vi "Controle_Manip_Main_GUI_WorkingBackup_211222.vi"() -> ()   [LabVIEW 2019] (continued)
                          frame #2 {
                            w3390 = T29."Enabled" ("Disabled")
                            n2748 = property on="Center Wavelength (nm)" class="DigNum (strict)"("DisabledEnum"=w3390) -> ()  [unwired: 2 in, 2 out]
                            n2749 = property on="Grating" class="CmbBox"("DisabledEnum"=w3390) -> ()  [unwired: 2 in, 2 out]
                            n2750 = property on="Exit mirror" class="Ring (strict)"("DisabledEnum"=w3390) -> ()  [unwired: 2 in, 2 out]
                          }
                        }
                      }
                      frame True {
                        n2751 = local write "LightField Automation error out"(w3391) -> ()
                        n2752 = local write "LightField Automation out"(w3392) -> ()
                      }
                    }
                  }
                }
              }
            }
          }
          event "Conv/Energy (eV)", "Conv/Wavelength (nm)", "Conv/Time (s)", "Conv/Wavenumber (m-1)": Value Change {
            n2753 = event-data() -> ("CtlRef"=w3395:refnum<vi>, "NewVal"=w3393:dbl)  [unwired: 1 in, 4 out]
            n2754 = property class="DigNum (strict)"(reference=w3395) -> ("Label.Text"=w3394:string)  [unwired: 1 in, 2 out]
            n2755 = case shown="\"Conv/Energy (eV)\"" w3394 {
              tunnel: w3393 -> [w3403 _ w3416 _]
              frame "Conv/Wavelength (nm)", Default {
                n2756 = Multiply(x=w3403, y=1e-09) -> (x*y=w3401:dbl)
                n2757 = Divide(x=1.0, y=w3401) -> (x/y=w3398:dbl)
                n2758 = Divide(x=w3401, y=299792458.0) -> (x/y=w3400:dbl)
                n2759 = Divide(x=w3398, y=100.0) -> (x/y=w3396:dbl)
                n2760 = Divide(x=1239.842, y=w3403) -> (x/y=w3405:dbl)
                n2761 = local write "Conv/Energy (eV)"(w3405) -> ()
                n2762 = local write "Conv/Wavenumber (m-1)"(w3396) -> ()
                n2763 = local write "Conv/Time (s)"(w3400) -> ()
              }
              frame "Conv/Time (s)" {
              }
              frame "Conv/Energy (eV)" {
                n2764 = Divide(x=1239.842, y=w3416) -> (x/y=w3415:dbl)
                n2765 = Multiply(x=w3415, y=1e-09) -> (x*y=w3412:dbl)
                n2766 = local write "Conv/Wavelength (nm)"(w3415) -> ()
                n2767 = Divide(x=1.0, y=w3412) -> (x/y=w3409:dbl)
                n2768 = Divide(x=w3409, y=100.0) -> (x/y=w3407:dbl)
                n2769 = Divide(x=w3412, y=299792458.0) -> (x/y=w3410:dbl)
                n2770 = local write "Conv/Wavenumber (m-1)"(w3407) -> ()
                n2771 = local write "Conv/Time (s)"(w3410) -> ()
              }
              frame "Conv/Wavenumber (m-1)" {
              }
            }
          }
          event "CCD ROI": Value Change {
            n2772 = event-data() -> ()  [unwired: 1 in, 6 out]
            n2773 = local read "LightField On?"() -> (w3418:bool)
            n2774 = case shown="True" w3418 {
              frame False {
              }
              frame True {
                n2775 = stacked-sequence {
                  frame #0 {
                    n2776 = property on="CCD ROI" class="Enum (strict)"("DisabledEnum"=T29."Disabled and Grayed Out" ("Disabled")) -> ()  [unwired: 2 in, 2 out]
                  }
                  frame #1 {
                    n2777 = local read "LightField Automation error out"() -> (w3422:errorcluster)
                    n2778 = local read "LightField Automation out"() -> (w3424:refnum<class "LightField Automation.lvclass">)
                    n2779 = local read "CCD ROI"() -> (w3423:T20)
                    n2780 = call "Adv_SetROI.vi"("error in (no error)"=w3422, "ROI"=w3423, "LightField Automation in"=w3424) -> ("error out"=w3421:errorcluster, "LightField Automation out"=w3420:refnum<class "LightField Automation.lvclass">)  [unwired: 7 in]
                    n2781 = local write "LightField Automation out"(w3420) -> ()
                    n2782 = local write "LightField Automation error out"(w3421) -> ()
                  }
                  frame #2 {
                    n2783 = property on="CCD ROI" class="Enum (strict)"("DisabledEnum"=T29."Enabled" ("Disabled")) -> ()  [unwired: 2 in, 2 out]
                  }
                }
              }
            }
          }
          event "Cryostat": Value Change {
            n2784 = event-data() -> ("NewVal"=w3426:enum16{"Montana", "Oxford"})  [unwired: 1 in, 5 out]
            n2785 = case shown="\"Montana\"" w3426 {
              frame "Oxford" {
                w3427 = FALSE
                n2786 = property on="FSM Up" class="Bool (strict)"("Visible"=w3427) -> ()  [unwired: 2 in, 2 out]
                n2787 = property on="FSM Left" class="Bool (strict)"("Visible"=w3427) -> ()  [unwired: 2 in, 2 out]
                n2788 = property on="FSM Axis Step" class="DigNum (strict)"("Visible"=w3427) -> ()  [unwired: 2 in, 2 out]
                n2789 = property on="FSM Down" class="Bool (strict)"("Visible"=w3427) -> ()  [unwired: 2 in, 2 out]
                n2790 = property on="FSM Right" class="Bool (strict)"("Visible"=w3427) -> ()  [unwired: 2 in, 2 out]
              }
              frame "Montana" {
                w3428 = TRUE
                n2791 = property on="FSM Up" class="Bool (strict)"("Visible"=w3428) -> ()  [unwired: 2 in, 2 out]
                n2792 = property on="FSM Left" class="Bool (strict)"("Visible"=w3428) -> ()  [unwired: 2 in, 2 out]
                n2793 = property on="FSM Axis Step" class="DigNum (strict)"("Visible"=w3428) -> ()  [unwired: 2 in, 2 out]
                n2794 = property on="FSM Down" class="Bool (strict)"("Visible"=w3428) -> ()  [unwired: 2 in, 2 out]
                n2795 = property on="FSM Right" class="Bool (strict)"("Visible"=w3428) -> ()  [unwired: 2 in, 2 out]
              }
            }
          }
          event "Excitation Power (uW)": Mouse Down; "Excitation Wavelength (nm)", "Excitation Source": Value Change {
            n2796 = event-data() -> ("CtlRef"=w3432:refnum<vi>)  [unwired: 1 in, 3 out]
            n2797 = property class="Num"(reference=w3432) -> ("Label.Text"=w3431:string)  [unwired: 1 in, 2 out]
            n2798 = case shown="\"Excitation Source\"" w3431 {
              tunnel: [w3433 w3434 w3445 w3470] -> w3429
              frame "False", Default {
                n2799 = local read "Excitation Wavelength (nm)"() -> (w3433:dbl)
              }
              frame "Excitation Power (uW)" {
                n2800 = local read "PM16-120 On?"() -> (w3435:bool)
                n2801 = case shown="True" w3435 {
                  tunnel: [w3436 w3437] -> w3434
                  frame False {
                    n2802 = local read "Excitation Wavelength (nm)"() -> (w3436:dbl)
                  }
                  frame True {
                    n2803 = local read "Excitation Wavelength (nm)"() -> (w3437:dbl)
                    n2804 = local read "Photodiode handle out"() -> (w3444:refnum<visa-resource-name>)
                    n2805 = local read "Photodiode error out"() -> (w3443:errorcluster)
                    n2806 = call <instrlib>:"TLPM Set Wavelength.vi"("error in (no error)"=w3443, "Wavelength (0.0)"=w3437, "instrument handle"=w3444) -> ("error out"=w3442:errorcluster, "instrument handle out"=w3441:refnum<visa-resource-name>)  [unwired: 7 in]
                    n2807 = call <instrlib>:"TLPM Measure Power.vi"("error in (no error)"=w3442, "instrument handle"=w3441) -> ("error out"=w3438:errorcluster, "Power"=w3440:dbl, "instrument handle out"=w3439:refnum<visa-resource-name>)  [unwired: 7 in]
                    n2808 = local write "Photodiode handle out"(w3439) -> ()
                    n2809 = local write "Photodiode error out"(w3438) -> ()
                    n2810 = local write "Excitation Power (uW)"(w3440) -> ()
                  }
                }
              }
              frame "Excitation Wavelength (nm)" {
                n2811 = stacked-sequence {
                  tunnel: [_ w3457] -> w3445
                  frame #0 {
                    n2812 = local read "Excitation Source"() -> (w3449:enum16{"P", "CW", "SK"})
                    n2813 = local read "LLTF On?"() -> (w3450:bool)
                    n2814 = Equal?(x=w3449, y=enum16{"P", "CW", "SK"}."SK") -> (x = y?=w3447:bool)
                    n2815 = And(x=w3450, y=w3447) -> (x .and. y?=w3446:bool)
                    n2816 = case shown="True" w3446 {
                      frame False {
                      }
                      frame True {
                        n2817 = local read "Excitation Wavelength (nm)"() -> (w3456:dbl)
                        n2818 = local read "LLTFDevice Interface"() -> (w3455:refnum<k7>)
                        n2819 = call "testmove.vi"("p_TargetWavelength"=w3456, "reference"=w3455) -> ("CurrentWavelength"=w3453:dbl, "CurrentAngle"=w3454:dbl, "Device reference out"=w3452:refnum<k7>, "Device moved"=w3451:bool)  [unwired: 4 in, 2 out]
                        n2820 = local write "LLTFDevice Interface"(w3452) -> ()
                        n2821 = local write "Device moved"(w3451) -> ()
                        n2822 = local write "CurrentAngle"(w3454) -> ()
                        n2823 = local write "CurrentWL"(w3453) -> ()
                      }
                    }
                  }
                  frame #1 {
                    n2824 = local read "PM16-120 On?"() -> (w3458:bool)
                    n2825 = case shown="True" w3458 {
                      tunnel: [w3459 w3460] -> w3457
                      frame False {
                        n2826 = local read "Excitation Wavelength (nm)"() -> (w3459:dbl)
                      }
                      frame True {
                        n2827 = local read "Excitation Wavelength (nm)"() -> (w3460:dbl)
                        n2828 = local read "Photodiode handle out"() -> (w3467:refnum<visa-resource-name>)
                        n2829 = local read "Photodiode error out"() -> (w3466:errorcluster)
                        n2830 = call <instrlib>:"TLPM Set Wavelength.vi"("error in (no error)"=w3466, "Wavelength (0.0)"=w3460, "instrument handle"=w3467) -> ("error out"=w3465:errorcluster, "instrument handle out"=w3464:refnum<visa-resource-name>)  [unwired: 7 in]
                        n2831 = call <instrlib>:"TLPM Measure Power.vi"("error in (no error)"=w3465, "instrument handle"=w3464) -> ("error out"=w3461:errorcluster, "Power"=w3463:dbl, "instrument handle out"=w3462:refnum<visa-resource-name>)  [unwired: 7 in]
                        n2832 = local write "Photodiode handle out"(w3462) -> ()
                        n2833 = local write "Photodiode error out"(w3461) -> ()
                        n2834 = local write "Excitation Power (uW)"(w3463) -> ()
                      }
                    }
                  }
                }
              }
              frame "Excitation Source" {
                n2835 = local read "Excitation Source"() -> (w3469:enum16{"P", "CW", "SK"})
                n2836 = local read "PM16-120 On?"() -> (w3471:bool)
                n2837 = case shown="Default" w3469 {
                  tunnel: [TRUE ("Laser on?") w3474] -> w3468
                  frame Default {
                  }
                  frame "CW" {
                    n2838 = local read "Laser on? Control"() -> (w3474:bool)
                    n2839 = local write "Excitation Wavelength (nm)"(448.5 ("Excitation Wavelength (nm)")) -> ()
                  }
                }
                n2840 = case shown="True" w3471 {
                  tunnel: [w3475 w3476] -> w3470
                  frame False {
                    n2841 = local read "Excitation Wavelength (nm)"() -> (w3475:dbl)
                  }
                  frame True {
                    n2842 = local read "Excitation Wavelength (nm)"() -> (w3476:dbl)
                    n2843 = local read "Photodiode handle out"() -> (w3483:refnum<visa-resource-name>)
                    n2844 = local read "Photodiode error out"() -> (w3482:errorcluster)
                    n2845 = call <instrlib>:"TLPM Set Wavelength.vi"("error in (no error)"=w3482, "Wavelength (0.0)"=w3476, "instrument handle"=w3483) -> ("error out"=w3481:errorcluster, "instrument handle out"=w3480:refnum<visa-resource-name>)  [unwired: 7 in]
                    n2846 = call <instrlib>:"TLPM Measure Power.vi"("error in (no error)"=w3481, "instrument handle"=w3480) -> ("error out"=w3477:errorcluster, "Power"=w3479:dbl, "instrument handle out"=w3478:refnum<visa-resource-name>)  [unwired: 7 in]
                    n2847 = local write "Photodiode handle out"(w3478) -> ()
                    n2848 = local write "Photodiode error out"(w3477) -> ()
                    n2849 = local write "Excitation Power (uW)"(w3479) -> ()
                  }
                }
                n2850 = local write "Laser on?"(w3468) -> ()
              }
            }
            n2851 = control-ref of="Laser on?"() -> (w3430:refnum<vi>)
            n2852 = call "ExcWL2LaserrColor.vi"("Wavelength (380 - 780)"=w3429, "Laser on?"=w3430) -> ()  [unwired: 1 in]
          }
          event "Exit mirror": Value Change {
            n2853 = event-data() -> ("NewVal"=w3484:u16)  [unwired: 1 in, 5 out]
            n2854 = local read "LightField On?"() -> (w3485:bool)
            n2855 = case shown="True" w3485 {
              tunnel: w3484 -> [_ w3492]
              frame False {
              }
              frame True {
                n2856 = stacked-sequence {
                  tunnel: w3492 -> [_ w3498 _]
                  tunnel: [_ w3497 _] -> w3487
                  tunnel: [_ w3496 _] -> w3486
                  frame #0 {
                    n2857 = control-ref of="Exit mirror"() -> (w3495:refnum<vi>)
                    n2858 = Build Array(w3495) -> (w3494:refnum<vi>[])
                    n2859 = call "Enable&Disable_Controls.vi"("Enum"=enum16{"Enabled", "Disabled", "Disabled&Grayed"}."Disabled&Grayed", "References"=w3494) -> ()  [unwired: 1 in]
                  }
                  frame #1 {
                    n2860 = case shown="4, Default" w3498 {
                      tunnel: [enum16{"Enabled", "Disabled", "Disabled&Grayed"}."Disabled&Grayed" ("Enum") enum16{"Enabled", "Disabled", "Disabled&Grayed"}."Enabled" ("Enum")] -> w3497
                      tunnel: [AcqMode."APD 1" ("Acq Mode") w3512] -> w3496
                      frame 5 {
                      }
                      frame 4, Default {
                        n2861 = property on="Acq Mode" class="Enum (strict)"() -> ("Value"=w3511:T3)  [unwired: 2 in, 2 out]
                        n2862 = Not Equal?(x=w3511, y=AcqMode."Image" ("Acq Mode")) -> (x != y?=w3509:bool)
                        n2863 = case shown="True" w3509 {
                          tunnel: [AcqMode."Image" ("Acq Mode") AcqMode."Spectrum" ("Acq Mode")] -> w3512
                          frame False {
                          }
                          frame True {
                          }
                        }
                      }
                    }
                    n2864 = local read "LightField Automation error out"() -> (w3506:errorcluster)
                    n2865 = local read "LightField Automation out"() -> (w3505:refnum<class "LightField Automation.lvclass">)
                    n2866 = call "spec_GetOpticalExitPort.vi"("error in (no error)"=w3506, "LightField Automation in"=w3505) -> ("error out"=w3503:errorcluster, "Exit Port Location"=w3502:T33, "LightField Automation out"=w3504:refnum<class "LightField Automation.lvclass">)  [unwired: 7 in]
                    n2867 = Equal?(x=w3502, y=w3498) -> (x = y?=w3501:bool)
                    n2868 = case shown="False" w3501 {
                      tunnel: w3504 -> [w3526 w3528]
                      tunnel: w3503 -> [w3525 w3527]
                      tunnel: w3498 -> [w3524 _]
                      tunnel: [w3517 w3528] -> w3500
                      tunnel: [w3516 w3527] -> w3499
                      frame False {
                        n2869 = call "spec_SetOpticalExitPort.vi"("error in (no error)"=w3525, "Exit Port Location"=w3524, "LightField Automation in"=w3526) -> ("error out"=w3519:errorcluster, "LightField Automation out"=w3518:refnum<class "LightField Automation.lvclass">)  [unwired: 7 in]
                        n2870 = call "spec_GetCenterWavelength.vi"("error in (no error)"=w3519, "LightField Automation in"=w3518) -> ("error out"=w3522:errorcluster, "Center Wavelength"=w3520:dbl, "LightField Automation out"=w3521:refnum<class "LightField Automation.lvclass">)  [unwired: 7 in]
                        n2871 = local write "Center Wavelength (nm)"(w3520) -> ()
                        n2872 = call "spec_getCalibration.vi"("error in (no error)"=w3522, "LightField Automation in"=w3521) -> ("error out"=w3516:errorcluster, "ColumnCalibration"=w3523:dbl[], "LightField Automation out"=w3517:refnum<class "LightField Automation.lvclass">)  [unwired: 7 in]
                        n2873 = local write "Wavelength calibration"(w3523) -> ()
                      }
                      frame True {
                      }
                    }
                    n2874 = local write "LightField Automation error out"(w3499) -> ()
                    n2875 = local write "LightField Automation out"(w3500) -> ()
                  }
                  frame #2 {
                    n2876 = property on="Exit mirror" class="Ring (strict)"() -> ("RingText.Text"=w3533:string)  [unwired: 2 in, 2 out]
                    n2877 = local read "Log file"() -> (w3537:string)
                    n2878 = control-ref of="Exit mirror"() -> (w3532:refnum<vi>)
                    n2879 = Concatenate Strings("Exit mirror set to " ("Add to log file"), w3533) -> (w3534:string)
                    n2880 = call "Write2LogFile.vi"("Add to log file"=w3534, "Log file before"=w3537, "Checkbox"=FALSE) -> ("Log file after"=w3536:string)
                    n2881 = Build Array(w3532) -> (w3531:refnum<vi>[])
                    n2882 = call "Enable&Disable_Controls.vi"("Enum"=enum16{"Enabled", "Disabled", "Disabled&Grayed"}."Enabled", "References"=w3531) -> ()  [unwired: 1 in]
                    n2883 = local write "Log file"(w3536) -> ()
                  }
                }
                n2884 = control-ref of="Accumulations"() -> (w3489:refnum<vi>)
                n2885 = control-ref of="CCD ROI"() -> (w3490:refnum<vi>)
                n2886 = control-ref of="Exposure Time (ms)"() -> (w3491:refnum<vi>)
                n2887 = Build Array(w3489, w3490, w3491) -> (w3488:refnum<vi>[])
                n2888 = call "Enable&Disable_Controls.vi"("Enum"=w3487, "References"=w3488) -> ()  [unwired: 1 in]
                n2889 = property on="Acq Mode" class="Enum (strict)"("Value"=w3486) -> ()  [unwired: 2 in, 2 out]
              }
            }
          }
          event "Exposure Time (ms)", "Acquire N: N": Value Change {
            n2890 = event-data() -> ("CtlRef"=w3541:refnum<vi>, "NewVal"=w3538:dbl)  [unwired: 1 in, 4 out]
            n2891 = property class="DigNum (strict)"(reference=w3541) -> ("Label.Text"=w3540:string)  [unwired: 1 in, 2 out]
            n2892 = local read "LightField On?"() -> (w3539:bool)
            n2893 = case shown="\"Exposure Time (ms)\"" w3540 {
              tunnel: w3538 -> [w3543 w3545]
              tunnel: w3539 -> [_ w3546]
              frame "Acquire N: N", Default {
                n2894 = local read "Acq Time (ms)"() -> (w3542:dbl)
                n2895 = call "unnecessary_multiplication.vi"("N"=w3543, "AcqTime ms"=w3542) -> ("AcqTime Total (s)"=w3544:dbl)
                n2896 = local write "Duration"(w3544) -> ()
              }
              frame "Exposure Time (ms)" {
                n2897 = case shown="True" w3546 {
                  tunnel: w3545 -> [_ w3558]
                  frame False {
                  }
                  frame True {
                    n2898 = local read "LightField Automation error out"() -> (w3565:errorcluster)
                    n2899 = local read "LightField Automation out"() -> (w3564:refnum<class "LightField Automation.lvclass">)
                    n2900 = Divide(x=w3558, y=1000.0) -> (x/y=w3559:dbl)
                    n2901 = call "Exp_CCD_GetExposureTime.vi"("error in (no error)"=w3565, "LightField Automation in"=w3564) -> ("error out"=w3560:errorcluster, "Exposure Time (s)"=w3563:dbl, "LightField Automation out"=w3561:refnum<class "LightField Automation.lvclass">)  [unwired: 7 in]
                    n2902 = Equal?(x=w3563, y=w3559) -> (x = y?=w3562:bool)
                    n2903 = case shown="False" w3562 {
                      tunnel: w3561 -> [w3568 w3578]
                      tunnel: w3560 -> [w3567 w3577]
                      tunnel: w3559 -> [w3569 _]
                      tunnel: w3558 -> [_ _]
                      frame False {
                        n2904 = stacked-sequence {
                          tunnel: w3569 -> [_ w3573 _]
                          tunnel: w3568 -> [_ w3572 _]
                          tunnel: w3567 -> [_ w3571 _]
                          frame #0 {
                            n2905 = property on="Exposure Time (ms)" class="DigNum (strict)"("DisabledEnum"=T29."Disabled and Grayed Out" ("Disabled")) -> ()  [unwired: 2 in, 2 out]
                          }
                          frame #1 {
                            n2906 = call "Exp_CCD_SetExposureTime.vi"("error in (no error)"=w3571, "Exposure Time (s)"=w3573, "LightField Automation in"=w3572) -> ("error out"=w3574:errorcluster, "LightField Automation out"=w3575:refnum<class "LightField Automation.lvclass">)  [unwired: 7 in]
                            n2907 = local write "LightField Automation out"(w3575) -> ()
                            n2908 = local write "LightField Automation error out"(w3574) -> ()
                          }
                          frame #2 {
                            n2909 = property on="Exposure Time (ms)" class="DigNum (strict)"("DisabledEnum"=T29."Enabled" ("Disabled")) -> ()  [unwired: 2 in, 2 out]
                          }
                        }
                      }
                      frame True {
                        n2910 = local write "LightField Automation out"(w3578) -> ()
                        n2911 = local write "LightField Automation error out"(w3577) -> ()
                      }
                    }
                  }
                }
                n2912 = disable-structure shown="Disabled" {
                  disable-tunnel: w3545 -> [w3552 _]
                  frame Disabled {
                    n2913 = local read "Scan Y Num. Pts"() -> (w3554:dbl)
                    n2914 = local read "Scan X Num. Pts"() -> (w3555:dbl)
                    n2915 = Divide(x=w3552, y=1000.0) -> (x/y=w3550:dbl)
                    n2916 = Multiply(x=w3554, y=w3555) -> (x*y=w3556:dbl)
                    n2917 = Add(x=w3550, y=0.17) -> (x+y=w3549:dbl)
                    n2918 = Multiply(x=w3549, y=w3556) -> (x*y=w3557:dbl)
                    n2919 = local write "Expected (s)"(w3557) -> ()
                  }
                  frame Enabled {
                  }
                }
                n2920 = local write "Acq Time (ms)"(w3545) -> ()
                n2921 = local read "Acquire N: N"() -> (w3547:dbl)
                n2922 = call "unnecessary_multiplication.vi"("N"=w3547, "AcqTime ms"=w3545) -> ("AcqTime Total (s)"=w3548:dbl)
                n2923 = local write "Duration"(w3548) -> ()
              }
            }
          }
          event "FSM Home": Mouse Down {
            n2924 = event-data() -> ()  [unwired: 1 in, 6 out]
            n2925 = local read "FSM 300 On?"() -> (w3579:bool)
            n2926 = case shown="True" w3579 {
              frame False {
              }
              frame True {
                w3581 = 0.0 ("Target Value (V)")
                w3580 = 0.0 ("Target Value (V)")
                n2927 = local read "FSM Y Task"() -> (w3582:refnum<k21>)
                n2928 = local read "FSM X Task"() -> (w3583:refnum<k21>)
                n2929 = call "FSMGoTo.vi"("Target Value (V)"=w3580, "FSM Task"=w3583) -> ()  [unwired: 1 out]
                n2930 = call "FSMGoTo.vi"("Target Value (V)"=w3581, "FSM Task"=w3582) -> ()  [unwired: 1 out]
                n2931 = local write "Scan X Readout (V)"(w3580) -> ()
                n2932 = local write "Scan Y Readout (V)"(w3581) -> ()
                n2933 = property on="XY Intensity Map" class="IntGraph (strict)"("Cursor.Cursor X"=w3580) -> ()  [unwired: 2 in, 2 out]
                n2934 = property on="XY Intensity Map" class="IntGraph (strict)"("Cursor.Cursor Y"=w3581) -> ()  [unwired: 2 in, 2 out]
              }
            }
          }
          event "FSM Up", "FSM Down", "FSM Left", "FSM Right": Mouse Down {
            n2935 = event-data() -> ("CtlRef"=w3585:refnum<vi>)  [unwired: 1 in, 7 out]
            n2936 = local read "FSM 300 On?"() -> (w3584:bool)
            n2937 = case shown="True" w3584 {
              tunnel: w3585 -> [_ w3590]
              frame False {
              }
              frame True {
                n2938 = property class="Bool (strict)"(reference=w3590) -> ("Label.Text"=w3588:string)  [unwired: 1 in, 2 out]
                n2939 = local read "FSM Axis Step"() -> (w3589:dbl)
                n2940 = case shown="\"FSM Down\"" w3588 {
                  tunnel: [w3594 w3598 w3602 w3606] -> w3587
                  tunnel: w3589 -> [w3592 w3596 w3600 w3604]
                  tunnel: [w3591 w3595 w3599 w3603] -> w3586
                  frame "FSM Up", Default {
                    n2941 = local read "Scan Y Readout (V)"() -> (w3593:dbl)
                    n2942 = Add(x=w3593, y=w3592) -> (x+y=w3591:dbl)
                    n2943 = local write "Scan Y Readout (V)"(w3591) -> ()
                    n2944 = property on="XY Intensity Map" class="IntGraph (strict)"("Cursor.Cursor Y"=w3591) -> ()  [unwired: 2 in, 2 out]
                    n2945 = local read "FSM Y Task"() -> (w3594:refnum<k21>)
                  }
                  frame "FSM Down" {
                    n2946 = local read "Scan Y Readout (V)"() -> (w3597:dbl)
                    n2947 = Subtract(x=w3597, y=w3596) -> (x-y=w3595:dbl)
                    n2948 = local write "Scan Y Readout (V)"(w3595) -> ()
                    n2949 = local read "FSM Y Task"() -> (w3598:refnum<k21>)
                    n2950 = property on="XY Intensity Map" class="IntGraph (strict)"("Cursor.Cursor Y"=w3595) -> ()  [unwired: 2 in, 2 out]
                  }
                  frame "FSM Left" {
                    n2951 = local read "Scan X Readout (V)"() -> (w3601:dbl)
                    n2952 = Subtract(x=w3601, y=w3600) -> (x-y=w3599:dbl)
                    n2953 = local write "Scan X Readout (V)"(w3599) -> ()
                    n2954 = property on="XY Intensity Map" class="IntGraph (strict)"("Cursor.Cursor X"=w3599) -> ()  [unwired: 2 in, 2 out]
                    n2955 = local read "FSM X Task"() -> (w3602:refnum<k21>)
                  }
                  frame "FSM Right" {
                    n2956 = local read "Scan X Readout (V)"() -> (w3605:dbl)
                    n2957 = Add(x=w3605, y=w3604) -> (x+y=w3603:dbl)
                    n2958 = local write "Scan X Readout (V)"(w3603) -> ()
                    n2959 = property on="XY Intensity Map" class="IntGraph (strict)"("Cursor.Cursor X"=w3603) -> ()  [unwired: 2 in, 2 out]
                    n2960 = local read "FSM X Task"() -> (w3606:refnum<k21>)
                  }
                }
                n2961 = call "FSMGoTo.vi"("Target Value (V)"=w3586, "FSM Task"=w3587) -> ()  [unwired: 1 out]
              }
            }
          }
          event "FSM X Axis Pos", "FSM Y Axis Pos": Value Change {
            # "Move steering mirror"
            n2962 = event-data() -> ("CtlRef"=w3609:refnum<vi>, "NewVal"=w3608:dbl)  [unwired: 1 in, 4 out]
            n2963 = local read "FSM 300 On?"() -> (w3607:bool)
            n2964 = case shown="True" w3607 {
              tunnel: w3609 -> [_ w3613]
              tunnel: w3608 -> [_ w3610]
              frame False {
              }
              frame True {
                n2965 = property class="DigNum (strict)"(reference=w3613) -> ("Label.Text"=w3612:string)  [unwired: 1 in, 2 out]
                n2966 = case shown="\"FSM Y Axis Pos\"" w3612 {
                  tunnel: [w3615 w3617] -> w3611
                  tunnel: w3610 -> [w3614 w3616]
                  frame "FSM Y Axis Pos" {
                    n2967 = local write "Scan Y Readout (V)"(w3614) -> ()
                    n2968 = property on="XY Intensity Map" class="IntGraph (strict)"("Cursor.Cursor Y"=w3614) -> ()  [unwired: 2 in, 2 out]
                    n2969 = local read "FSM Y Task"() -> (w3615:refnum<k21>)
                  }
                  frame "FSM X Axis Pos", Default {
                    n2970 = local write "Scan X Readout (V)"(w3616) -> ()
                    n2971 = property on="XY Intensity Map" class="IntGraph (strict)"("Cursor.Cursor X"=w3616) -> ()  [unwired: 2 in, 2 out]
                    n2972 = local read "FSM X Task"() -> (w3617:refnum<k21>)
                  }
                }
                n2973 = call "FSMGoTo.vi"("Target Value (V)"=w3610, "FSM Task"=w3611) -> ()  [unwired: 1 out]
              }
            }
          }
          event "Add location": Mouse Down {
            (unwired) FALSE
            w3620 = "\r"
            n2974 = event-data() -> ()  [unwired: 1 in, 8 out]
            n2975 = local read "Map Marker X Pos"() -> (w3624:i8)
            n2976 = local read "Map Marker Y Pos"() -> (w3625:i8)
            n2977 = Format Into String(w3624) -> (resulting string=w3623:string)  [unwired: 3 in, 1 out]
            n2978 = Format Into String(w3625) -> (resulting string=w3621:string)  [unwired: 3 in, 1 out]
            n2979 = Concatenate Strings(w3620, "### Location ", w3623, "x" ("string"), w3621, w3620) -> (w3619:string)
            n2980 = call "Write2Markdown.vi"("String"=w3619) -> ()
            "ExportMapPosition?" <- FALSE ("ExportMapPosition?")
          }
          event "Full scale": Value Change {
            n2981 = event-data() -> ()  [unwired: 1 in, 6 out]
            n2982 = stacked-sequence {
              frame #0 {
                w3635 = 1239.842
                n2983 = property on="CCD 1D Spectrum Main" class="XYGraph (strict)"() -> ("Value"=w3630:cluster{dbl[], dbl[]})  [unwired: 2 in, 2 out]
                n2984 = Unbundle(w3630) -> (w3629:dbl[])  [unwired: 1 out]
                n2985 = property on="CCD 1D Spectrum Main" class="XYGraph (strict)"("XScale.ScaleFit"=u8 1 ("X Scale.Scale Fit"), "YScale.Minimum"=0.0 ("Y Scale.Range:Minimum")) -> ("XScale.Minimum"=w3627:dbl, "XScale.Maximum"=w3632:dbl)  [unwired: 2 in, 2 out]
                n2986 = call "myMax.vi"("Array"=w3629) -> ("myMax"=w3628:dbl)  [unwired: 1 in]
                n2987 = Divide(x=w3635, y=w3627) -> (x/y=w3633:dbl)
                n2988 = Divide(x=w3635, y=w3632) -> (x/y=w3634:dbl)
                n2989 = property on="CCD 1D Spectrum Main" class="XYGraph (strict)"("YScale.Maximum"=w3628) -> ()  [unwired: 2 in, 2 out]
                n2990 = property on="CCD 1D Spectrum Main Energy Scale" class="XYGraph (strict)"("XScale.Maximum"=w3633, "XScale.Minimum"=w3634) -> ()  [unwired: 2 in, 2 out]
              }
              frame #1 {
                n2991 = property on="Full scale" class="Bool (strict)"("Value"=FALSE ("Full scale")) -> ()  [unwired: 2 in, 2 out]
              }
            }
          }
          event "Grating": Value Change {
            n2992 = event-data() -> ("NewVal"=w3639:string)  [unwired: 1 in, 5 out]
            n2993 = local read "LightField On?"() -> (w3638:bool)
            n2994 = case shown="True" w3638 {
              tunnel: w3639 -> [_ w3646]
              frame False {
              }
              frame True {
                n2995 = local read "LightField Automation error out"() -> (w3645:errorcluster)
                n2996 = local read "LightField Automation out"() -> (w3643:refnum<class "LightField Automation.lvclass">)
                n2997 = call "spec_GetGratings.vi"("error in (no error)"=w3645, "LightField Automation in"=w3643) -> ("error out"=w3644:errorcluster, "Current Grating"=w3641:string, "LightField Automation out"=w3642:refnum<class "LightField Automation.lvclass">)  [unwired: 6 in, 1 out]
                n2998 = Equal?(x=w3646, y=w3641) -> (x = y?=w3640:bool)
                n2999 = case shown="False" w3640 {
                  tunnel: w3646 -> [w3652 _]
                  tunnel: w3644 -> [w3651 w3678]
                  tunnel: w3642 -> [w3650 w3679]
                  frame False {
                    n3000 = stacked-sequence {
                      seq-local: [_ w3662 _ _ _] -> [_ _ w3667 _ _]
                      seq-local: [_ w3661 _ _ _] -> [_ _ w3666 _ _]
                      seq-local: [_ w3660 _ _ _] -> [_ _ w3663 _ _]
                      seq-local: [_ _ w3665 _ _] -> [_ _ _ w3675 _]
                      seq-local: [_ _ w3664 _ _] -> [_ _ _ w3674 _]
                      seq-local: [_ _ w3663 _ _] -> [_ _ _ w3672 _]
                      tunnel: w3650 -> [_ w3662 _ _ _]
                      tunnel: w3651 -> [_ w3661 _ _ _]
                      tunnel: w3652 -> [_ w3660 _ _ _]
                      tunnel: [_ _ _ w3675 _] -> w3657
                      tunnel: [_ _ _ w3674 _] -> w3656
                      frame #0 {
                        n3001 = property on="Grating" class="CmbBox"("DisabledEnum"=T29."Disabled and Grayed Out" ("Disabled")) -> ()  [unwired: 2 in, 2 out]
                      }
                      frame #1 {
                      }
                      frame #2 {
                        n3002 = call "spec_SetGrating.vi"("error in (no error)"=w3666, "GratingSelected"=w3663, "LightField Automation in"=w3667) -> ("error out"=w3664:errorcluster, "LightField Automation out"=w3665:refnum<class "LightField Automation.lvclass">)  [unwired: 7 in]
                      }
                      frame #3 {
                        n3003 = local read "Log file"() -> (w3671:string)
                        n3004 = Concatenate Strings("Grating changed to " ("string"), w3672) -> (w3670:string)
                        n3005 = call "Write2LogFile.vi"("Add to log file"=w3670, "Log file before"=w3671, "Checkbox"=FALSE) -> ("Log file after"=w3669:string)
                        n3006 = local write "Log file"(w3669) -> ()
                      }
                      frame #4 {
                        n3007 = property on="Background substract" class="Enum (strict)"("Val(Sgnl)"=enum16{"None", "Shutter"}."Shutter" ("Value (Signaling)")) -> ()  [unwired: 2 in, 2 out]
                        n3008 = property on="Grating" class="CmbBox"("DisabledEnum"=T29."Enabled" ("Disabled")) -> ()  [unwired: 2 in, 2 out]
                      }
                    }
                    n3009 = call "spec_GetCenterWavelength.vi"("error in (no error)"=w3656, "LightField Automation in"=w3657) -> ("error out"=w3655:errorcluster, "Center Wavelength"=w3653:dbl, "LightField Automation out"=w3654:refnum<class "LightField Automation.lvclass">)  [unwired: 7 in]
                    n3010 = local write "Center Wavelength (nm)"(w3653) -> ()
                    n3011 = local write "Background taken?"(FALSE ("Background taken?")) -> ()
                    n3012 = call "spec_getCalibration.vi"("error in (no error)"=w3655, "LightField Automation in"=w3654) -> ("error out"=w3649:errorcluster, "ColumnCalibration"=w3658:dbl[], "LightField Automation out"=w3648:refnum<class "LightField Automation.lvclass">)  [unwired: 7 in]
                    n3013 = local write "LightField Automation out"(w3648) -> ()
                    n3014 = local write "LightField Automation error out"(w3649) -> ()
                    n3015 = local write "Wavelength calibration"(w3658) -> ()
                  }
                  frame True {
                    n3016 = local write "LightField Automation out"(w3679) -> ()
                    n3017 = local write "LightField Automation error out"(w3678) -> ()
                  }
                }
              }
            }
          }
          event "Mono2 On": Value Change {
            n3018 = event-data() -> ("NewVal"=w3681:bool)  [unwired: 1 in, 5 out]
            n3019 = local read "ESP 300 On?"() -> (w3680:bool)
            n3020 = case shown="True" w3680 {
              tunnel: w3681 -> [_ w3682]
              frame False {
              }
              frame True {
                n3021 = case shown="True" w3682 {
                  frame False {
                    n3022 = stacked-sequence {
                      frame #0 {
                        n3023 = local read "ESP300 COM Port"() -> (w3686:refnum<visa-resource-name>)
                        n3024 = local read "ESP300 Error"() -> (w3687:errorcluster)
                        n3025 = call "Motor Off.vi"("error in (no error)"=w3687, "Axis"=1, "VISA resource name in"=w3686) -> ("error out"=w3684:errorcluster, "VISA resource name out"=w3683:refnum<visa-resource-name>)  [unwired: 7 in]
                        n3026 = local write "ESP300 Error"(w3684) -> ()
                        n3027 = local write "ESP300 COM Port"(w3683) -> ()
                      }
                      frame #1 {
                        n3028 = local read "Log file"() -> (w3690:string)
                        n3029 = call "Write2LogFile.vi"("Add to log file"="Mono2 motor turned off", "Log file before"=w3690, "Checkbox"=FALSE) -> ("Log file after"=w3691:string)
                        n3030 = local write "Log file"(w3691) -> ()
                      }
                    }
                  }
                  frame True {
                    n3031 = stacked-sequence {
                      frame #0 {
                        n3032 = local read "ESP300 COM Port"() -> (w3695:refnum<visa-resource-name>)
                        n3033 = local read "ESP300 Error"() -> (w3696:errorcluster)
                        n3034 = call "Motor On.vi"("error in (no error)"=w3696, "Axis"=1, "VISA resource name in"=w3695) -> ("error out"=w3693:errorcluster, "VISA resource name out"=w3692:refnum<visa-resource-name>)  [unwired: 7 in]
                        n3035 = local write "ESP300 Error"(w3693) -> ()
                        n3036 = local write "ESP300 COM Port"(w3692) -> ()
                      }
                      frame #1 {
                        n3037 = local read "Log file"() -> (w3699:string)
                        n3038 = call "Write2LogFile.vi"("Add to log file"="Mono2 motor turned on", "Log file before"=w3699, "Checkbox"=FALSE) -> ("Log file after"=w3700:string)
                        n3039 = local write "Log file"(w3700) -> ()
                      }
                    }
                  }
                }
              }
            }
          }
          event "Motor LinT On?", "Motor RotStage Exc On?", "Motor RotStage Det On?", "LinTFine Motor On?": Mouse Down {
            n3040 = event-data() -> ("CtlRef"=w3703:refnum<vi>)  [unwired: 1 in, 7 out]
            n3041 = property class="Bool (strict)"(reference=w3703) -> ("Label.Text"=w3702:string, "Value"=w3701:bool)  [unwired: 1 in, 2 out]
            n3042 = case shown="\"LinTFine Motor On?\"" w3702 {
              tunnel: w3701 -> [w3705 _ w3713 w3721 w3729]
              frame "Motor RotStage Exc On?" {
                n3043 = local read "ESP 301 On?"() -> (w3704:bool)
                n3044 = case shown="True" w3704 {
                  tunnel: w3705 -> [_ w3706]
                  frame False {
                  }
                  frame True {
                    n3045 = local read "ESP 301 COM Port"() -> (w3711:refnum<visa-resource-name>)
                    n3046 = local read "ESP 301 Error"() -> (w3710:errorcluster)
                    n3047 = call "Enable Disable Motor.vi"("error in (no error)"=w3710, "Action (F - OFF)"=w3706, "Axis (1)"=2, "VISA resource name"=w3711) -> ("error out"=w3708:errorcluster, "VISA resource name out"=w3709:refnum<visa-resource-name>)  [unwired: 2 in]
                    n3048 = local write "ESP 301 COM Port"(w3709) -> ()
                    n3049 = local write "ESP 301 Error"(w3708) -> ()
                  }
                }
              }
              frame Default {
                # "default do nothing"
              }
              frame "LinTFine Motor On?" {
                n3050 = local read "PZC200 On?"() -> (w3712:bool)
                n3051 = case shown="True" w3712 {
                  tunnel: w3713 -> [_ w3716]
                  frame False {
                  }
                  frame True {
                    n3052 = case shown="False" w3716 {
                      tunnel: ["1MF" "1MO" ("Command")] -> w3715
                      frame False {
                      }
                      frame True {
                      }
                    }
                    n3053 = local read "PZC200 Instrument Channel"() -> (w3717:string)
                    n3054 = call "SendCommand.vi"("Command"=w3715, "Instrument Channel"=w3717) -> ("Instrument Channel out"=w3714:string)  [unwired: 8 in, 1 out]
                    n3055 = local write "PZC200 Instrument Channel"(w3714) -> ()
                  }
                }
              }
              frame "Motor LinT On?" {
                n3056 = local read "ESP 301 On?"() -> (w3720:bool)
                n3057 = case shown="True" w3720 {
                  tunnel: w3721 -> [_ w3724]
                  frame False {
                  }
                  frame True {
                    n3058 = local read "ESP 301 COM Port"() -> (w3727:refnum<visa-resource-name>)
                    n3059 = local read "ESP 301 Error"() -> (w3726:errorcluster)
                    n3060 = call "Enable Disable Motor.vi"("error in (no error)"=w3726, "Action (F - OFF)"=w3724, "Axis (1)"=1, "VISA resource name"=w3727) -> ("error out"=w3722:errorcluster, "VISA resource name out"=w3723:refnum<visa-resource-name>)  [unwired: 2 in]
                    n3061 = local write "ESP 301 COM Port"(w3723) -> ()
                    n3062 = local write "ESP 301 Error"(w3722) -> ()
                  }
                }
              }
              frame "Motor RotStage Det On?" {
                n3063 = local read "ESP 301 On?"() -> (w3728:bool)
                n3064 = case shown="True" w3728 {
                  tunnel: w3729 -> [_ w3730]
                  frame False {
                  }
                  frame True {
                    n3065 = local read "ESP 301 COM Port"() -> (w3735:refnum<visa-resource-name>)
                    n3066 = local read "ESP 301 Error"() -> (w3734:errorcluster)
                    n3067 = call "Enable Disable Motor.vi"("error in (no error)"=w3734, "Action (F - OFF)"=w3730, "Axis (1)"=3, "VISA resource name"=w3735) -> ("error out"=w3732:errorcluster, "VISA resource name out"=w3733:refnum<visa-resource-name>)  [unwired: 2 in]
                    n3068 = local write "ESP 301 COM Port"(w3733) -> ()
                    n3069 = local write "ESP 301 Error"(w3732) -> ()
                  }
                }
              }
            }
          }
          event "PZC Position Readout (usteps)", "RotStage Exc Angle Readout (°)", "RotStage Det Angle Readout (°)", "Newport Linear Translation Stage Position Readout (mm)": Mouse Down {
            n3070 = event-data() -> ("CtlRef"=w3738:refnum<vi>)  [unwired: 1 in, 7 out]
            n3071 = property class="DigNum (strict)"(reference=w3738) -> ("Label.Text"=w3737:string)  [unwired: 1 in, 2 out]
            n3072 = case shown="\"RotStage Det Angle Readout (°)\"" w3737 {
              tunnel: [0.0 ("Position (units)") w3740 w3751 w3762 w3769] -> w3736
              frame "False", Default {
              }
              frame "RotStage Exc Angle Readout (°)" {
                n3073 = local read "ESP 301 On?"() -> (w3741:bool)
                n3074 = case shown="True" w3741 {
                  tunnel: [0.0 ("Position (units)") w3748] -> w3740
                  frame False {
                  }
                  frame True {
                    w3743 = 3 ("Axis (1)")
                    n3075 = local read "ESP 301 COM Port"() -> (w3746:refnum<visa-resource-name>)
                    n3076 = local read "ESP 301 Error"() -> (w3747:errorcluster)
                    n3077 = call "Read absolute position.vi"("error in (no error)"=w3747, "Axis (1)"=w3743, "VISA resource name"=w3746) -> ("error out"=w3744:errorcluster, "VISA resource name out"=w3745:refnum<visa-resource-name>)  [unwired: 2 in, 1 out]
                    n3078 = call "Read absolute position.vi"("error in (no error)"=w3744, "Axis (1)"=w3743, "VISA resource name"=w3745) -> ("error out"=w3749:errorcluster, "Position (units)"=w3748:dbl, "VISA resource name out"=w3750:refnum<visa-resource-name>)  [unwired: 2 in]
                    n3079 = local write "ESP 301 COM Port"(w3750) -> ()
                    n3080 = local write "RotStage Exc Angle Readout (°)"(w3748) -> ()
                    n3081 = local write "ESP 301 Error"(w3749) -> ()
                  }
                }
              }
              frame "RotStage Det Angle Readout (°)" {
                n3082 = local read "ESP 301 On?"() -> (w3752:bool)
                n3083 = case shown="True" w3752 {
                  tunnel: [0.0 ("Position (units)") w3759] -> w3751
                  frame False {
                  }
                  frame True {
                    w3754 = 2 ("Axis (1)")
                    n3084 = local read "ESP 301 COM Port"() -> (w3755:refnum<visa-resource-name>)
                    n3085 = local read "ESP 301 Error"() -> (w3758:errorcluster)
                    n3086 = call "Read absolute position.vi"("error in (no error)"=w3758, "Axis (1)"=w3754, "VISA resource name"=w3755) -> ("error out"=w3757:errorcluster, "VISA resource name out"=w3756:refnum<visa-resource-name>)  [unwired: 2 in, 1 out]
                    n3087 = call "Read absolute position.vi"("error in (no error)"=w3757, "Axis (1)"=w3754, "VISA resource name"=w3756) -> ("error out"=w3761:errorcluster, "Position (units)"=w3759:dbl, "VISA resource name out"=w3760:refnum<visa-resource-name>)  [unwired: 2 in]
                    n3088 = local write "ESP 301 COM Port"(w3760) -> ()
                    n3089 = local write "RotStage Det Angle Readout (°)"(w3759) -> ()
                    n3090 = local write "ESP 301 Error"(w3761) -> ()
                  }
                }
              }
              frame "Newport Linear Translation Stage Position Readout (mm)" {
                n3091 = local read "ESP 301 On?"() -> (w3763:bool)
                n3092 = case shown="True" w3763 {
                  tunnel: [0.0 ("Position (units)") w3768] -> w3762
                  frame False {
                  }
                  frame True {
                    n3093 = local read "ESP 301 COM Port"() -> (w3766:refnum<visa-resource-name>)
                    n3094 = local read "ESP 301 Error"() -> (w3765:errorcluster)
                    n3095 = call "Read Actual Position.vi"("error in (no error)"=w3765, "Axis (1)"=1, "VISA resource name"=w3766) -> ("Position (units)"=w3768:dbl)  [unwired: 2 in, 2 out]
                    n3096 = local write "Newport Linear Translation Stage Position Readout (mm)"(w3768) -> ()
                  }
                }
              }
              frame "PZC Position Readout (usteps) " {
                n3097 = local read "PZC200 On?"() -> (w3770:bool)
                n3098 = case shown="True" w3770 {
                  tunnel: [0 ("Position") w3772] -> w3769
                  frame False {
                  }
                  frame True {
                    n3099 = local read "PZC200 Instrument Channel"() -> (w3775:string)
                    n3100 = call "PZCGetPos.vi"("Instrument Channel"=w3775) -> ("Instrument Channel Out"=w3773:string, "Position"=w3772:i32, "error out"=w3774:errorcluster)  [unwired: 1 in]
                    n3101 = local write "PZC Error"(w3774) -> ()
                    n3102 = local write "PZC Position Readout (usteps)"(w3772) -> ()
                    n3103 = local write "PZC200 Instrument Channel"(w3773) -> ()
                  }
                }
              }
            }
            "Position (units)" <- w3736
          }
          event "Reset origins": Value Change {
            n3104 = event-data() -> ("NewVal"=w3776:bool)  [unwired: 1 in, 5 out]
            n3105 = case shown="True" w3776 {
              frame False {
              }
              frame True {
                n3106 = disable-structure shown="Disabled" {
                  frame Disabled {
                    n3107 = local read "PZC Position Readout (usteps)"() -> ()  [unwired: 1 out]
                    n3108 = local read "Newport Linear Translation Stage Position Readout (mm)"() -> ()  [unwired: 1 out]
                  }
                  frame Enabled {
                  }
                }
              }
            }
          }
          event "RotStage Exc Angle (°)", "RotStage Det Angle (°)", "Newport Linear Translation Stage Position (mm)", "Newport PZA12 Stage Position (usteps)": Value Change {
            n3109 = event-data() -> ("CtlRef"=w3779:refnum<vi>, "NewVal"=w3778:dbl)  [unwired: 1 in, 4 out]
            n3110 = property class="DigNum (strict)"(reference=w3779) -> ("Label.Text"=w3777:string)  [unwired: 1 in, 2 out]
            n3111 = case shown="\"RotStage Exc Angle (°)\"" w3777 {
              tunnel: w3777 -> [_ _ w3798 _ w3838 w3867]
              tunnel: w3778 -> [_ w3781 w3797 w3833 w3837 w3866]
              frame "False", Default {
              }
              frame "Newport PZA12 Stage Position (usteps)" {
                n3112 = local read "PZC200 On?"() -> (w3780:bool)
                n3113 = case shown="True" w3780 {
                  tunnel: w3781 -> [_ w3783]
                  frame False {
                  }
                  frame True {
                    n3114 = local read "PZC200 Instrument Channel"() -> (w3787:string)
                    n3115 = call "PZCGetPos.vi"("Instrument Channel"=w3787) -> ("Instrument Channel Out"=w3784:string, "Position"=w3786:i32)  [unwired: 1 in, 1 out]
                    n3116 = Not Equal?(x=w3783, y=w3786) -> (x != y?=w3785:bool)
                    n3117 = case shown="True" w3785 {
                      tunnel: w3784 -> [w3788 w3791]
                      tunnel: w3783 -> [_ w3790]
                      tunnel: [w3788 w3789] -> w3782
                      frame False {
                      }
                      frame True {
                        n3118 = stacked-sequence {
                          tunnel: w3791 -> [w3795]
                          tunnel: w3790 -> [w3794]
                          tunnel: [w3792] -> w3789
                          frame #0 {
                            n3119 = call "PZC_MoveAbs.vi"("Target"=w3794, "Instrument"=w3795) -> ("Final Position"=w3793:i32, "Instrument out"=w3792:string)  [unwired: 1 in, 1 out]
                            n3120 = local write "PZC Position Readout (usteps)"(w3793) -> ()
                          }
                        }
                      }
                    }
                    n3121 = local write "PZC200 Instrument Channel"(w3782) -> ()
                  }
                }
              }
              frame "Newport Linear Translation Stage Position (mm)" {
                n3122 = local read "ESP 301 On?"() -> (w3796:bool)
                n3123 = case shown="True" w3796 {
                  tunnel: w3798 -> [_ w3813]
                  tunnel: w3797 -> [_ w3802]
                  frame False {
                  }
                  frame True {
                    n3124 = case shown="\"Newport Linear Translation Stage Position (mm)\"" w3813 {
                      tunnel: [2 1 3] -> w3814
                      tunnel: [w3817 w3820 w3823] -> w3811
                      tunnel: w3802 -> [w3816 w3819 w3822]
                      frame "RotStage Det Angle (°)" {
                        n3125 = local write "RotStage Det Angle (°)"(w3816) -> ()
                        n3126 = control-ref of="RotStage Det Angle Readout (°)"() -> (w3817:refnum<vi>)
                      }
                      frame "Newport Linear Translation Stage Position (mm)" {
                        n3127 = control-ref of="Newport Linear Translation Stage Position Readout (mm)"() -> (w3820:refnum<vi>)
                        n3128 = local write "Newport Linear Translation Stage Position (mm)"(w3819) -> ()
                      }
                      frame "RotStage Exc Angle (°)", Default {
                        n3129 = local write "RotStage Exc Angle (°)"(w3822) -> ()
                        n3130 = control-ref of="RotStage Exc Angle Readout (°)"() -> (w3823:refnum<vi>)
                      }
                    }
                    n3131 = local read "Excitation Wavelength (nm)"() -> (w3807:dbl)
                    n3132 = local read "Photodiode Status"() -> (w3799:bool)
                    n3133 = local read "Photodiode handle out"() -> (w3809:refnum<visa-resource-name>)
                    n3134 = local read "Photodiode error out"() -> (w3808:errorcluster)
                    n3135 = local read "ESP 301 Error"() -> (w3815:errorcluster)
                    n3136 = control-ref of="Excitation Power (uW)"() -> (w3810:refnum<vi>)
                    n3137 = call <instrlib>:"TLPM Set Wavelength.vi"("error in (no error)"=w3808, "Wavelength (0.0)"=w3807, "instrument handle"=w3809) -> ("error out"=w3805:errorcluster, "instrument handle out"=w3806:refnum<visa-resource-name>)  [unwired: 7 in]
                    n3138 = local read "ESP 301 COM Port"() -> (w3801:refnum<visa-resource-name>)
                    n3139 = call "Go2Angle.vi"("VISA resource name"=w3801, "Photodiode"=w3806, "RotStage Det Angle Readout (°) 4"=w3811, "Excitation Power (uW) 2"=w3810, "Photodiode on?"=w3799, "Axis ESP301 / RotStage"=w3814, "ESP301 Error"=w3815, "Photodiode error"=w3805, "Position (units)"=w3802) -> ("Photodiode out"=w3803:refnum<visa-resource-name>, "VISA resource name out"=w3800:refnum<visa-resource-name>, "Photodiode"=w3804:errorcluster, "ESP301 Error out"=w3812:errorcluster)  [unwired: 3 in]
                    n3140 = local write "ESP 301 Error"(w3812) -> ()
                    n3141 = local write "Photodiode handle out"(w3803) -> ()
                    n3142 = local write "Photodiode error out"(w3804) -> ()
                    n3143 = local write "ESP 301 COM Port"(w3800) -> ()
                  }
                }
              }
              frame "Newport Linear Translation Stage Position (mm) Test" {
                w3828 = 1 ("Axis (1)")
                n3144 = local read "ESP 301 COM Port"() -> (w3832:refnum<visa-resource-name>)
                n3145 = local read "ESP 301 Error"() -> (w3831:errorcluster)
                n3146 = call "Move Absolute.vi"("error in (no error)"=w3831, "Position (0 units)"=w3833, "Axis (1)"=w3828, "VISA resource name"=w3832) -> ("error out"=w3834:errorcluster, "VISA resource name out"=w3835:refnum<visa-resource-name>)  [unwired: 2 in]
                n3147 = call "Wait For Motion Stop.vi"("error in (no error)"=w3834, "Axis (0)"=w3828, "VISA resource name"=w3835) -> ("error out"=w3829:errorcluster, "VISA resource name out"=w3830:refnum<visa-resource-name>)  [unwired: 3 in]
                n3148 = call "Read absolute position.vi"("error in (no error)"=w3829, "Axis (1)"=w3828, "VISA resource name"=w3830) -> ("error out"=w3826:errorcluster, "Position (units)"=w3825:dbl, "VISA resource name out"=w3827:refnum<visa-resource-name>)  [unwired: 2 in]
                n3149 = local write "Newport Linear Translation Stage Position Readout (mm)"(w3825) -> ()
                n3150 = local write "ESP 301 COM Port"(w3827) -> ()
                n3151 = local write "ESP 301 Error"(w3826) -> ()
              }
              frame "RotStage Exc Angle (°)" {
                n3152 = local read "ESP 301 On?"() -> (w3836:bool)
                n3153 = case shown="True" w3836 {
                  tunnel: w3838 -> [_ w3855]
                  tunnel: w3837 -> [_ w3854]
                  frame False {
                  }
                  frame True {
                    n3154 = case shown="\"RotStage Exc Angle (°)\", Default" w3855 {
                      tunnel: [2 1 3] -> w3851
                      tunnel: [w3857 w3860 w3863] -> w3848
                      tunnel: w3854 -> [w3856 w3859 w3862]
                      frame "RotStage Det Angle (°)" {
                        n3155 = local write "RotStage Det Angle (°)"(w3856) -> ()
                        n3156 = control-ref of="RotStage Det Angle Readout (°)"() -> (w3857:refnum<vi>)
                      }
                      frame "Newport Linear Translation Stage Position (mm)" {
                        n3157 = control-ref of="Newport Linear Translation Stage Position Readout (mm)"() -> (w3860:refnum<vi>)
                        n3158 = local write "Newport Linear Translation Stage Position (mm)"(w3859) -> ()
                      }
                      frame "RotStage Exc Angle (°)", Default {
                        n3159 = local write "RotStage Exc Angle (°)"(w3862) -> ()
                        n3160 = control-ref of="RotStage Exc Angle Readout (°)"() -> (w3863:refnum<vi>)
                      }
                    }
                    n3161 = local read "Excitation Wavelength (nm)"() -> (w3844:dbl)
                    n3162 = local read "Photodiode handle out"() -> (w3846:refnum<visa-resource-name>)
                    n3163 = local read "Photodiode error out"() -> (w3845:errorcluster)
                    n3164 = local read "Photodiode Status"() -> (w3839:bool)
                    n3165 = local read "ESP 301 Error"() -> (w3852:errorcluster)
                    n3166 = control-ref of="Excitation Power (uW)"() -> (w3847:refnum<vi>)
                    n3167 = call <instrlib>:"TLPM Set Wavelength.vi"("error in (no error)"=w3845, "Wavelength (0.0)"=w3844, "instrument handle"=w3846) -> ("error out"=w3842:errorcluster, "instrument handle out"=w3843:refnum<visa-resource-name>)  [unwired: 7 in]
                    n3168 = local read "ESP 301 COM Port"() -> (w3853:refnum<visa-resource-name>)
                    n3169 = call "Go2Angle.vi"("VISA resource name"=w3853, "Photodiode"=w3843, "RotStage Det Angle Readout (°) 4"=w3848, "Excitation Power (uW) 2"=w3847, "Photodiode on?"=w3839, "Axis ESP301 / RotStage"=w3851, "ESP301 Error"=w3852, "Photodiode error"=w3842, "Position (units)"=w3854) -> ("Photodiode out"=w3840:refnum<visa-resource-name>, "VISA resource name out"=w3850:refnum<visa-resource-name>, "Photodiode"=w3841:errorcluster, "ESP301 Error out"=w3849:errorcluster)  [unwired: 3 in]
                    n3170 = local write "Photodiode error out"(w3841) -> ()
                    n3171 = local write "ESP 301 Error"(w3849) -> ()
                    n3172 = local write "ESP 301 COM Port"(w3850) -> ()
                    n3173 = local write "Photodiode handle out"(w3840) -> ()
                  }
                }
              }
              frame "RotStage Det Angle (°)" {